vi "Hysteresis-CorrectionData.vi"(6 "path":path, 7 "hypothesis":T1(ring)=enum."middle", 8 "Picture Parameters (to save)":cluster{"Width":dbl, "Height":dbl}={"Width"=0.000136, "Height"=0.000136}, 9 "rel Range":dbl=1.0 format="%#_13g", 10 "Frame":bool=TRUE, 11 "Raw 2":cluster{"fwd":dbl[][], "bwd":dbl[][]}={"fwd"=array512x512[262144 elements], "bwd"=array512x512[262144 elements]}) -> (1 "Preisach":dbl[](array[numeric]), 2 "Polynomial Coefficients":cluster{"fwd":dbl[], "bwd":dbl[]}, 3 "Corrected":cluster{"fwd":dbl[][], "bwd":dbl[][]}, 4 "final covariance":dbl, 5 "initial covariance":dbl)   [LabVIEW 2016]
uses:
  libgwyscan-1.2-labview2015-win32/controls/parameters for save Gwyddion arrays.ctl
panel:
  out "Fwd - Bwd Corrected":dbl[][](graph)
  out "Raw":cluster{"fwd":dbl[][], "bwd":dbl[][]}
  out "hysteresis loop":cluster{dbl[], dbl[]}[](graph)
  out "deleted pixels":i32 caption="pixel to delete (left of fwd and right of bwd)"
  out "image without way":dbl[][](graph)
  # "Insert 2 images (Trace/Retrace), chose an hypothesis and the part of the piezo used (1=full range, 0.5=half range)"
  # "This returns:\n-corrected images\n-hysteresis of the X piezo (Preisach + 2 3rd order polynoms)\n-phase delay (in pixel)"
  # "Polynomial coefficients"
  # "Raw"
  # "Corrected"
  # "Substraction after correction"
  # "x^0"
  # "x^1"
  # "x^2"
  # "x^3"
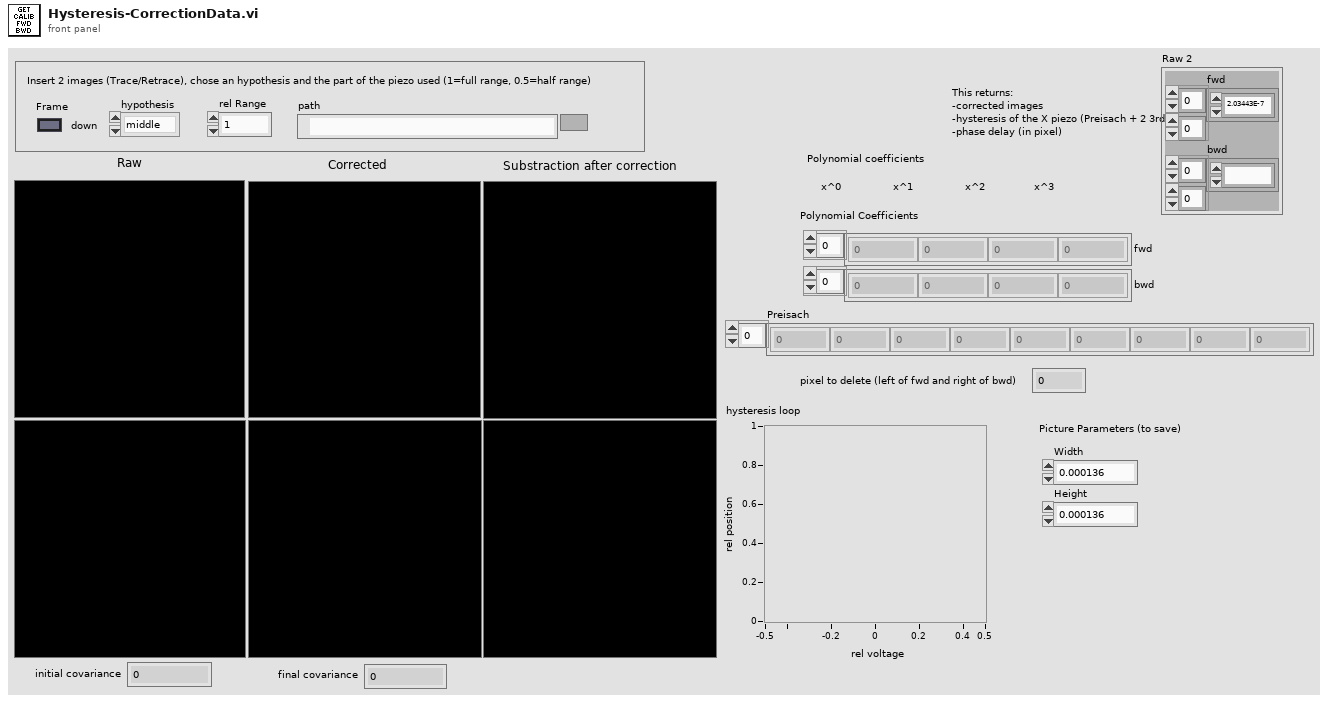
[diagram p1: front panel]
types:
  T1 = enum16{"bwd", "middle", "fwd", "linear", "2nd esti"}
  T2 = typedef "parameters for save Gwyddion arrays.ctl" = cluster{"X res":i32, "Y res ":i32, "xreal":dbl, "yreal":dbl, "nChannels":i32, "filename":string, "Descriptions":string[], "xyunit":string[], "Z unit":string[]}
  T3 = cluster{"Polynomial Coefficients fwd":dbl[], "Polynomial Coefficients bwd":dbl[]}
  T4 = cluster{"After Correction data":dbl[][], "After Correction data":dbl[][]}
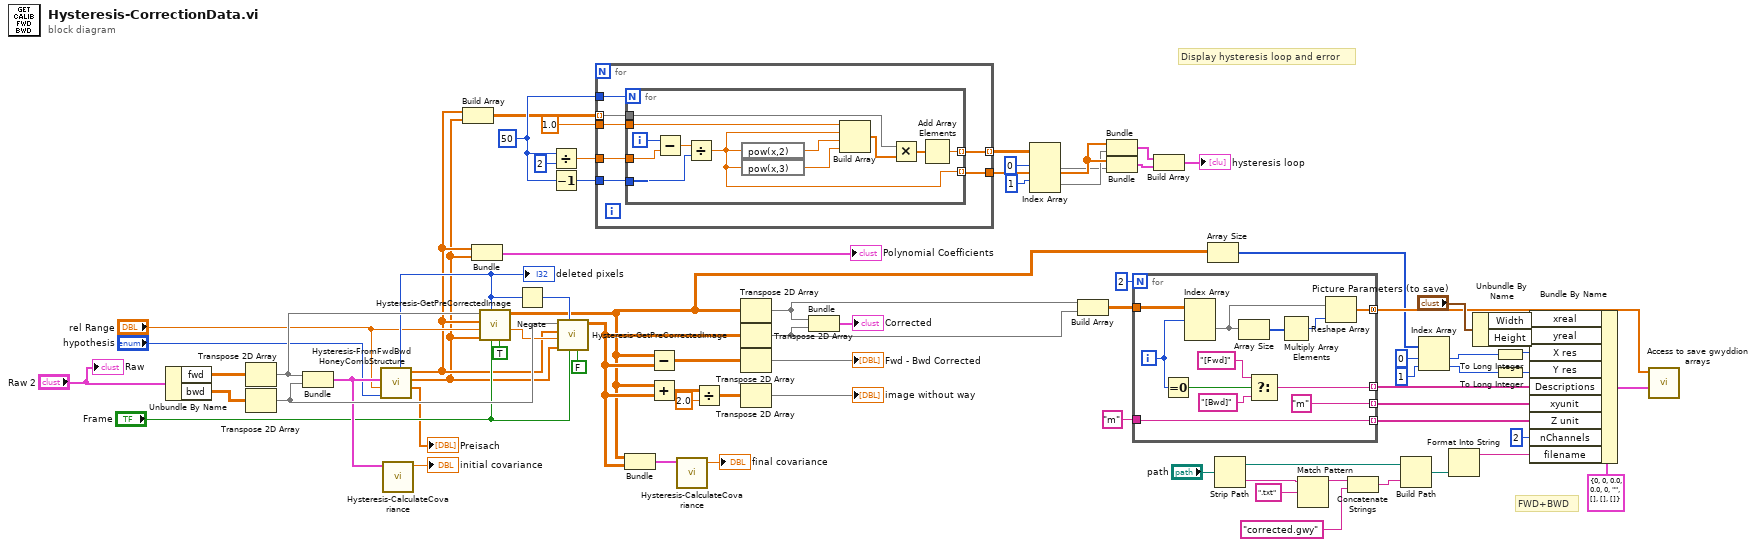
[diagram p0: block diagram]
diagram:
  w71 = 50
  # "FWD+BWD"
  # "Display hysteresis loop and error"
  n1 = Unbundle By Name("Raw 2") -> ("fwd"=w53:dbl[][], "bwd"=w52:dbl[][])
  n2 = Transpose 2D Array(2D array=w53) -> (transposed array=w73:dbl[][])
  n3 = Transpose 2D Array(2D array=w52) -> (transposed array=w75:dbl[][])
  n4 = Bundle(w73, w75) -> (w74:cluster{dbl[][], dbl[][]})  [unwired: 1 in]
  n5 = call "Hysteresis-FromFwdBwdHoneyCombStructure.vi"("hypothesis"="hypothesis", "relative Range"="rel Range", "Pictures"=w74) -> ("Preisach"=→"Preisach":dbl[], "Polynomial Coefficients bwd"=w37:dbl[], "Polynomial Coefficients fwd"=w49:dbl[], "pixel to delete"=w57:i32)  [unwired: 4 in, 1 out]
  "deleted pixels" <- w57
  n6 = call "Hysteresis-CalculateCovariance.vi"("Pictures"=w74) -> ("covariance"=→"initial covariance":dbl)  [unwired: 10 in]
  n7 = Build Array(w49, w37) -> (w48:dbl[][])
  n8 = Bundle("Polynomial Coefficients fwd"=w49, "Polynomial Coefficients bwd"=w37) -> (→"Polynomial Coefficients":T3)  [unwired: 1 in]
  n9 = call "Hysteresis-GetPreCorrectedImage.vi"("fwd?"=TRUE, "frame up?"="Frame", "pixel to delete"=w57, "Polynomial Coefficients bwd"=w37, "Relative Range"="rel Range", "Polynomial Coefficients fwd"=w49, "Before Correction Data"=w73) -> ("After Correction data"=w2:dbl[][])  [unwired: 4 in]
  n10 = Negate(x=w57) -> (-x=w51:i32)
  n11 = Divide(x=w71, y=2) -> (x/y=w69:dbl)
  n12 = Decrement(x=w71) -> (x-1=w68:i32)
  n13 = call "Hysteresis-GetPreCorrectedImage.vi"("fwd?"=FALSE, "frame up?"="Frame", "pixel to delete"=w51, "Polynomial Coefficients bwd"=w37, "Relative Range"="rel Range", "Polynomial Coefficients fwd"=w49, "Before Correction Data"=w75) -> ("After Correction data"=w41:dbl[][])  [unwired: 4 in]
  n14 = for {
    tunnel: w71 -> [w82]
    tunnel: w69 -> [w81]
    tunnel: w68 -> [w80]
    tunnel: [w79] -> w64
    tunnel: 1.0 ("element") -> [w78]
    tunnel: w48 -> [w77] mode=indexing
    tunnel: [w76] -> w47 mode=indexing
    n15 = for {
      N: w82 -> [_]
      tunnel: w81 -> [w93]
      tunnel: w80 -> [w90]
      tunnel: [w87] -> w79 mode=indexing
      tunnel: w78 -> [w91]
      tunnel: w77 -> [w85]
      tunnel: [w83] -> w76 mode=indexing
      i -> [w94]
      n16 = Subtract(x=w94, y=w93) -> (x-y=w92:dbl)
      n17 = Divide(x=w92, y=w90) -> (x/y=w87:dbl)
      n18 = expression code="pow(x,2)"(w87) -> (w88:dbl)
      n19 = expression code="pow(x,3)"(w87) -> (w89:dbl)
      n20 = Build Array(w91, w87, w88, w89) -> (w84:dbl[])
      n21 = Multiply(x=w85, y=w84) -> (x*y=w86:dbl[])
      n22 = Add Array Elements(numeric array=w86) -> (sum=w83:dbl)
    }
  }
  n23 = Bundle("After Correction data"=w2, "After Correction data"=w41) -> (w58:T4)  [unwired: 1 in]
  n24 = Subtract(x=w2, y=w41) -> (x-y=w36:dbl[][])
  n25 = Add(x=w2, y=w41) -> (x+y=w39:dbl[][])
  n26 = call "Hysteresis-CalculateCovariance.vi"("Pictures"=w58) -> ("covariance"=→"final covariance":dbl)  [unwired: 10 in]
  n27 = Divide(x=w39, y=2.0) -> (x/y=w38:dbl[][])
  n28 = Transpose 2D Array(2D array=w2) -> (transposed array=w1:dbl[][])
  n29 = Transpose 2D Array(2D array=w41) -> (transposed array=w6:dbl[][])
  n30 = Transpose 2D Array(2D array=w36) -> (transposed array=→"Fwd - Bwd Corrected":dbl[][])
  n31 = Transpose 2D Array(2D array=w38) -> (transposed array=→"image without way":dbl[][])
  n32 = Bundle(w1, w6) -> (→"Corrected":cluster{dbl[][], dbl[][]})  [unwired: 1 in]
  n33 = Index Array(array=w47, index (row) #1=0 ("index (row)"), index (row) #2=1 ("index (row)")) -> (element #1=w43:dbl[], element #2=w44:dbl[])  [unwired: 2 in]
  n34 = Build Array(w1, w6) -> (w18:dbl[][][])
  n35 = Bundle(w64, w44) -> (w65:cluster{dbl[], dbl[]})  [unwired: 1 in]
  n36 = Bundle(w64, w43) -> (w66:cluster{dbl[], dbl[]})  [unwired: 1 in]
  n37 = for {
    N: 2 -> [_]
    tunnel: w18 -> [w106]
    tunnel: [w103] -> w13 mode=concatenating
    tunnel: [w96] -> w12 mode=indexing
    tunnel: ["m"] -> w11 mode=indexing
    tunnel: [w98] -> w10 mode=indexing
    tunnel: "m" -> [w98]
    i -> [w97]
    n38 = Equal To 0?(x=w97) -> (x = 0?=w101:bool)
    n39 = Index Array(array=w106, index (dim 0)=w97) -> (element=w104:dbl[][])  [unwired: 2 in]
    n40 = Array Size(array=w104) -> (size(s)=w95:i32[])
    n41 = Select(t="[Fwd]", s=w101, f="[Bwd]") -> (s? t:f=w96:string)
    n42 = Multiply Array Elements(1:w95) -> (0:w105:i32)
    n43 = Reshape Array(w104, w105) -> (w103:dbl[])
  }
  n44 = Build Array(w65, w66) -> (→"hysteresis loop":cluster{dbl[], dbl[]}[])
  n45 = Array Size(array=w2) -> (size(s)=w5:i32[])
  n46 = Strip Path(path="path") -> (stripped path=w25:path, name=w31:string)
  n47 = Match Pattern(string=w31, regular expression=".txt") -> (before substring=w33:string)  [unwired: 1 in, 3 out]
  n48 = Concatenate Strings(w33, "corrected.gwy" ("filename")) -> (w23:string)
  n49 = Build Path(base path=w25, name or relative path=w23) -> (appended path=w21:path)
  n50 = Index Array(array=w5, index #1=0 ("index"), index #2=1 ("index")) -> (element #1=w29:i32, element #2=w30:i32)
  n51 = Format Into String(w21) -> (resulting string=w22:string)  [unwired: 3 in, 1 out]
  n52 = Unbundle By Name("Picture Parameters (to save)") -> ("Width"=w9:dbl, "Height"=w8:dbl)
  n53 = To Long Integer(number=w29) -> (32bit integer=w14:i32)
  n54 = To Long Integer(number=w30) -> (32bit integer=w15:i32)
  n55 = Bundle By Name(cluster=T2 {"X res"=0, "Y res "=0, "xreal"=0.0, "yreal"=0.0, "nChannels"=0, "filename"="", "Descriptions"=[], "xyunit"=[], "Z unit"=[]} ("parameters for save Gwyddion arrays"), "xreal"=w9, "yreal"=w8, "X res"=w14, "Y res"=w15, "Descriptions"=w12, "xyunit"=w11, "Z unit"=w10, "nChannels"=2 ("y"), "filename"=w22) -> (w17:T2)
  n56 = call "Access to save gwyddion arrays.vi"("parameters for save Gwyddion arrays"=w17, "data IN"=w13) -> ()  [unwired: 3 in, 1 out]
  "Raw" <- "Raw 2"
